vi "UHR-Fleezers Control (host) - 12.3.1.vi"() -> ()   [LabVIEW 2012] (continued)
  T20 = cluster{"New Image":T2, "New Image":T2, "New Image":T2, "New Image":T2, "New Image":T2}
  T21 = typedef "XDNodeRunTimeDep.lvlib/timing_clust.ctl" = cluster{"Expected End [f-1]":u64, "Actual End [f-1]":u64, "Finished Late? [f-1]":bool, "Expected End [i-1]":u64, "Actual End [i-1]":u64, "Finished Late? [i-1]":bool, "Expected Start [i]":u64, "Actual Start [i]":u64, "Expected Start [f]":u64, "Actual Start [f]":u64, "Source Name":string, "Structure Name":string, "Period":i64, "Deadline":i64, "Offset":i64, "Start":i64, "Priority":i32, "Timeout":i32, "Mode":T22, "Wakeup Reason":T23, "Error":errorcluster, "Source Type":string, "Secondary Source Type":string, "Global End Time":u64, "Global Start Time":u64, "Frame Duration":u64, "Iteration Duration":u64, "Assigned CPU":i32, "I/O Scan Engine Mode":u32}
  T22 = typedef "XDNodeRunTimeDep.lvlib/nitl_modes.ctl" = enum32{"No Change", "Process missed periods, maintain original phase", "Discard missed periods, maintain original phase", "Process missed periods, ignore original phase", "Discard missed periods, ignore original phase"}
  T23 = typedef "XDNodeRunTimeDep.lvlib/wakeup.ctl" = enum32{"Normal", "Aborted", "Asynchronous wakeup", "Timing source error", "Timed loop error", "Timeout"}
  T24 = enum32{"Status", "Sample Stage", "Syringe Pump", "Trap Control (RF)", "APD Counting", "Fluorescence Laser Control", "Trap AI", "Video", "FPGA"}
  T25 = enum16{"big-endian, network order", "native, host order", "little-endian"}
  T26 = enum16{"open", "replace", "create", "open or create", "replace or create", "replace or create with confirmation"}
  T27 = cluster{"Scan Range AOD (nm) 2":dbl, "Step Size AOD (nm) 2":dbl, "Scan Speed AOD (nm/s) 2":dbl, "Number of scans (AOD) 2":u16, "Label":string}
  T28 = cluster{"[0]":dbl, "[1]":dbl, "[2]":dbl, "[3]":dbl, "[4]":dbl, "[5]":dbl}
  T29 = cluster{"Diameter (mm)":dbl, "Units":dbl, "Volume":dbl, "Rate":dbl}
  T30 = cluster{"Left":i32, "Top":i32, "Width":u32, "Height":u32}
  T31 = cluster{cluster{"Left":i32, "Top":i32, "Width":u32, "Height":u32}}[]
  T32 = enum32{"Normal Display", "Dual Display (APD)", "FFT", "High Res Display"}
  T33 = cluster{"Origin Pixel":cluster{"X":sgl, "Y":sgl}, "Angle Relative to Horizontal (deg)":sgl, "Axis Reference":u32}
  T34 = typedef "Simple Grid Descriptor" = cluster{"X Step":sgl, "Y Step":sgl, "Unit":T35}
  T35 = typedef "Image Unit" = enum32{"Undefined", "Angström", "Micrometer", "Millimeter", "Centimeter", "Meter", "Kilometer", "Microinch", "Inch", "Feet", "Nautical miles", "Standard miles", "Steps"}
  T36 = cluster{"averaging mode":u16, "weighting mode":u16, "number of averages":u32}
  T37 = cluster{"dB On (F)":bool, "unwrap phase (F)":bool, "convert to degree (F)":bool}
  T38 = cluster{string, string, string, string, string, string, string, string}
  T39 = cluster{string, string, string, string, string, string, string, string, string, string, string, string}
  T40 = cluster{string, string, string, string, string, string, string, string, string, string, string, string, string}
  T41 = cluster{string, string, string, string, string, string, string, string, string, string, string, string, string, string}
  T42 = cluster{"BD 1 Frequency 1 (MHz)":dbl, "BD 1 Frequency 2 (MHz)":dbl}
  T43 = cluster{"f0":dbl, "df":dbl, "magnitude":dbl[]}[][]
  T44 = enum32{"setting", "request", "request control", "info", "statistics", "system settings", "I/O sub system", "HRT control", "camera descriptions", "device specific data", "event sub system settings", "event sub system results", "image memory manager"}
  T45 = typedef "AviRefnum.ctl" = refnum<k1>
  T46 = typedef "imagedata.ctl" = cluster{"image type":i32, "image depth":i32, "image":u8[], "mask":u8[], "colors":u32[], "Rectangle":cluster{"left":i16, "top":i16, "right":i16, "bottom":i16}}
diagram:
  w69 = u16 20 items=["1.0"=10, "1.5"=15, "2.0"=20] ("stop bits (10: 1 bit)")
  w72 = u16 20 items=["1.0"=10, "1.5"=15, "2.0"=20] ("stop bits (10: 1 bit)")
  w98 = u16 20 items=["1.0"=10, "1.5"=15, "2.0"=20] ("stop bits (10: 1 bit)")
  w4 = T17 2 items=["Grayscale (U8)", "Grayscale (I16)", "Grayscale (SGL)", "Complex (CSG)", "RGB (U32)", "HSL (U32)", "RGB (U64)", "Grayscale (U16)"] ("Image Type")
  w228 = 10.0 ("y")
  w227 = 32767.0 ("y")
  w243 = 6.0  # clock mult.
  w244 = 49152000.0  # TCXO frequ.
  # "What are these?"
  # "I don't think you need to do this.\nEverytime you want to adjust phase you always set this anyway.\nSince we removed the separate +/- controls.\n\nHaven't added for added fl lasers.  Should remove this code."
  # "Bottom 1 Harvard"
  # "Top 3 Harvard"
  # "Center Harvard"
  # "Bottom 1 Harvard"
  # "Top 3 Harvard"
  # "Center Harvard"
  n1 = Build Array("DIO count 1 (ticks)", "DIO count 2 (ticks)", "DIO count 3 (ticks)") -> (w149:u16[])
  n2 = xnode "Open FPGA VI Reference"("resource name"=T18 "750kHzDAQ") -> ("FPGA VI Reference Out"=w252:T19, "error out"=w251:errorcluster)  [unwired: 1 in]
  n3 = local read "AO1"() -> (w222:dbl)
  n4 = local read "AO2"() -> (w221:dbl)
  n5 = local read "Scan Increment (MHz)"() -> (w239:dbl)
  n6 = local read "Continuous MCL Scanning"() -> (w209:bool)
  n7 = local read "Fast Scan Dir"() -> (w208:bool)
  n8 = xnode "Invoke Method"("FPGA VI Reference In"=w252, "error in"=w251) -> ("FPGA VI Reference Out"=w8:T19, "error out"=w168:errorcluster)
  n9 = local read "Number of scans (MCL)"() -> (w210:u64)
  n10 = Multiply(x=w222, y=w227) -> (x*y=w224:dbl)
  n11 = Multiply(x=w221, y=w227) -> (x*y=w226:dbl)
  n12 = Divide(x=w224, y=w228) -> (x/y=w223:dbl)
  n13 = Divide(x=w226, y=w228) -> (x/y=w225:dbl)
  n14 = To Word Integer(number=w223) -> (16bit integer=w220:i16)
  n15 = To Word Integer(number=w225) -> (16bit integer=w219:i16)
  n16 = Not(x=w208) -> (.not. x?=w203:bool)
  n17 = local read "Cycles/step (MCL)"() -> (w211:u64)
  n18 = Multiply(x=w239, y=1000.0) -> (x*y=w246:dbl)
  n19 = local read "Scan steps (MCL)"() -> (w212:u64)
  n20 = local read "Desired Scan Incr (V)"() -> (w214:dbl)
  n21 = Scale By Power Of 2(n=48, x=w246) -> (x*2^n=w247:dbl)
  n22 = Unbundle By Name(cluster{"output high":i16, "output low":i16} {"output high"=3000, "output low"=0} ("FB output range 1")) -> ("output high"=w50:i16, "output low"=w49:i16)
  n23 = Multiply(x=w244, y=w243) -> (x*y=w242:dbl)
  n24 = Divide(x=w247, y=w242) -> (x/y=w241:dbl)
  n25 = local read "Setpoints (V)"() -> (w258:cluster{"Set 1":dbl, "Set 2":dbl})
  n26 = To Quad Integer(1:w241) -> (0:w238:i64)
  n27 = Divide(x=40000000.0, y="AI Count (ticks)") -> (x/y=w199:dbl)
  n28 = Multiply(x=w214, y=32767.0) -> (x*y=w216:dbl)
  n29 = local read "Trap Intensity PID Gains"() -> (w253:T9)
  n30 = local write "Trap Pos FIFO Timeout"(u16 0 ("Trap Pos FIFO Timeout")) -> ()
  n31 = local read "Number Interlace Sets"() -> (w142:u8)
  n32 = Split 1D Array(array=w149, index=w142) -> (first subarray=w151:u16[])  [unwired: 1 out]
  n33 = Add Array Elements(numeric array=w151) -> (sum=w150:u16)
  n34 = local read "# Samples/channel"() -> (w231:u32)
  n35 = local read "Number of F/B Scans (AOD)"() -> (w232:u16)
  n36 = local read "Not-Interlacing Set"() -> (w141:enum32{"Set 1", "Set 2", "Set 3"})
  n37 = To Unsigned Byte Integer(number=w141) -> (unsigned 8bit integer=w147:u8)
  n38 = Index Array(array=w149, index=w147) -> (element=w148:u16)
  n39 = local read "Feedback On/Off"() -> (w261:cluster{"Set 1":bool, "Set 2":bool})
  n40 = local read "Scan steps (AOD)"() -> (w237:u64)
  n41 = local read "All FB On/Off"() -> (w262:bool)
  n42 = local read "Cycles/step (AOD)"() -> (w236:u64)
  n43 = local write "AI rate (Hz)"(w199) -> ()
  n44 = Divide(x=w216, y=10.0) -> (x/y=w215:dbl)
  n45 = Multiply(x=w237, y=w236) -> (x*y=w235:u64)
  n46 = Unbundle By Name(w253) -> ("proportional gain (Kc)"=w54:i16, "integral gain (Kc*Ts/Ti)"=w53:i16, "derivative gain (Kc*Td/Ts)"=w52:i16)
  n47 = property on="AI Count (ticks)" class="DigNum (strict)"("Val(Sgnl)"="AI Count (ticks)") -> ()  [unwired: 2 in, 2 out]
  n48 = Multiply(x=3276.7, y=w258) -> (x*y=w257:cluster{"Set 1":dbl, "Set 2":dbl})
  n49 = To Word Integer(number=w215) -> (16bit integer=w213:i16)
  n50 = Multiply(x=w235, y=u64 2) -> (x*y=w233:u64)
  n51 = Divide(x=w199, y="FPGA Ave.") -> (x/y=w200:dbl)
  n52 = To Word Integer(number=w257) -> (16bit integer=w256:cluster{"Set 1":i16, "Set 2":i16})
  n53 = Multiply(x=w233, y=w232) -> (x*y=w230:u64)
  n54 = local read "Sets to FIFO (Traps)"() -> (w58:T15)
  n55 = local write "Ave. Rate (Hz)"(w200) -> ()
  n56 = Divide(x=w230, y=w231) -> (x/y=w229:dbl)
  n57 = Unbundle By Name(w256) -> ("Set 1"=w255:i16, "Set 2"=w254:i16)
  n58 = local read "2D or 1D Scan"() -> (w160:bool)
  n59 = local write "Data points/scans"(w230) -> ()
  n60 = local read "Scan BD"() -> (w248:bool)
  n61 = And(x=w261, y=w262) -> (x .and. y?=w260:cluster{"Set 1":bool, "Set 2":bool})
  n62 = local write "Data points/scan (f/b)"(w233) -> ()
  n63 = Reciprocal(x=w200) -> (1/x=w201:dbl)
  n64 = local read "N Acq Sets (Traps + Fl.)"() -> (w192:i16)
  n65 = local write "N sets should be saved"(w229) -> ()
  n66 = Unbundle By Name(w260) -> ("Set 1"=w264:bool, "Set 2"=w263:bool)
  n67 = local read "Interlace"() -> (w143:bool)
  n68 = Select(t=w150, s=w143, f=w148) -> (s? t:f=w140:u16)
  n69 = local write "Update Count (MCL)"(w140) -> ()
  n70 = local write "Total Counts (ticks)"(w140) -> ()
  n71 = local write "Ave. Period (s)"(w201) -> ()
  n72 = Unbundle By Name(w58) -> ("Set 1"=w57:bool, "Set 2"=w56:bool, "Set 3"=w55:bool)
  n73 = property on="2D or 1D Scan" class="Bool (strict)"("Val(Sgnl)"=w160) -> ()  [unwired: 2 in, 2 out]
  n74 = xnode "Read/Write Control"("FPGA VI Reference In"=w159, "error in"=w168, "ai count"="AI Count (ticks)", "Interlace ON/OFF"=w143, "Number Interlace Cycles"=w142, "Set 1"=w57, "Set 2"=w56, "Set 3"=w55, "FB On/Off Set 1"=w264, "FB On/Off Set 2"=w263, "Interlace Off Parameters"=w141, "FB Setpoint Set 1"=w255, "FB Setpoint Set 2"=w254, "P1"=w54, "I1"=w53, "D1"=w52, "FB1 output high"=w50, "FB1 output low"=w49, "Cycles per step"=w236, "Scan BD"=w248, "Number of scans"=w232, "Scan steps"=w237, "Scan freq.  increment"=w238, "AO1"=w220, "AO2"=w219, "Scan freq.  increment (MCL)"=w213, "Scan steps (MCL)"=w212, "Cycles per step (MCL)"=w211, "Number of scans (MCL)"=w210, "MCL count"=w140, "Cont. Scan (MCL)"=w209, "MCL Scan Axis"=w203, "1D or 2D Scan?"=w160, "N of AI1 Int Acq Sets"=w192, "Amp switch delay"="Amp switch delay", "Swap F1 and F2"="Swap F1 and F2", "APD to FIFO"=FALSE, "DIO count 1 (ticks)"="DIO count 1 (ticks)", "DIO count 2 (ticks)"="DIO count 2 (ticks)", "DIO count 3 (ticks)"="DIO count 3 (ticks)") -> ("FPGA VI Reference Out"=w10:T19, "error out"=w9:errorcluster)  [unwired: 1 in]
  n75 = local read "Laser interlacing mode"() -> (w139:enum32{"Laser ON", "Laser OFF", "Interlace"})
  n76 = local read "Green Laser ON"() -> (w138:bool)
  n77 = local read "Trap Pos. FB Range"() -> (w48:T12)
  n78 = local read "Trap Pos. FB Gains"() -> (w47:T11)
  n79 = Multiply(x="Green Intensity - FB OFF (%)", y=655.35) -> (x*y=w131:dbl)
  n80 = local read "Invert laser interlacing"() -> (w25:bool)
  n81 = local read "Trap Pos. AI1 X Pre-scale"() -> (w86:u16)
  n82 = Multiply(x="Green FB Setpoint (mV)", y=3.2767) -> (x*y=w128:dbl)
  n83 = local read "Trap Pos FB Int Count"() -> (w80:u16)
  n84 = local read "Differential FB?"() -> (w74:bool)
  n85 = local read "Neg. TTrig FPGA"() -> (w76:bool)
  n86 = Multiply(x="Red FB Setpoint (mV)", y=3.2767) -> (x*y=w34:dbl)
  n87 = To Unsigned Word Integer(number=w131) -> (unsigned 16bit integer=w129:u16)
  n88 = Multiply(x="Red Intensity - FB OFF (%)", y=655.35) -> (x*y=w30:dbl)
  n89 = To Word Integer(number=w128) -> (16bit integer=w126:i16)
  n90 = Unbundle By Name("Green FB Gains") -> ("proportional gain (Kc)"=w39:i16, "integral gain (Kc*Ts/Ti)"=w38:i16, "derivative gain (Kc*Td/Ts)"=w37:i16)
  n91 = case shown="False" w138 {
    tunnel: w139 -> [_ w290]
    tunnel: [enum32{"Laser ON", "Laser OFF", "Interlace"}."Laser OFF" ("Green laser mode") w290] -> w24
    frame False {
    }
    frame True {
    }
  }
  n92 = To Word Integer(number=w34) -> (16bit integer=w31:i16)
  n93 = Unbundle By Name("Red FB Gains") -> ("proportional gain (Kc)"=w22:i16, "integral gain (Kc*Ts/Ti)"=w21:i16, "derivative gain (Kc*Td/Ts)"=w20:i16)
  n94 = Unbundle By Name(w47) -> ("proportional gain (Kc)"=w43:fxp<+/-,16,8>, "integral gain (Kc*Ts/Ti)"=w42:fxp<+/-,16,8>, "derivative gain (Kc*Td/Ts)"=w41:fxp<+/-,16,8>)
  n95 = To Unsigned Word Integer(number=w30) -> (unsigned 16bit integer=w27:u16)
  n96 = Unbundle By Name(w48) -> ("output high"=w46:fxp<+/-,16,1>, "output low"=w44:fxp<+/-,16,1>)
  n97 = local read "Trap Pos FB Monitor\nT1 or T2"() -> (w91:bool)
  n98 = local read "Trap Pos FB Negate Action"() -> (w90:bool)
  n99 = local read "Trap Pos. FB Offset Factor"() -> (w89:i64)
  n100 = local read "Trap Pos. FB Mult Factor"() -> (w88:i64)
  n101 = xnode "Read/Write Control"("FPGA VI Reference In"=w10, "error in"=w9, "Invert GI 2"=w25, "Operating Mode 2"=w24, "P3"=w39, "I3"=w38, "D3"=w37, "Green FB Setpoint"=w126, "Green FB On/Off"="Green FB On/Off", "Current Out"=w129, "Green int current ON count adj"="Green int current ON count adj", "Operating Mode"=w24, "Invert GI"=w25, "Trap Pos FB Monitor T1 or T2"=w91, "Trap Pos FB Negate Action"=w90, "Trap Pos. FB Offset Factor"=w89, "Trap Pos. FB Mult Factor"=w88, "Force feedback"=FALSE, "AI1 X Scale"=w86, "Trap Pos to FIFO"=TRUE, "Trap Pos FB Int Count"=w80, "TTrig Negate Pos"=w76, "FB Trig Integrate"="FB Trig Integrate", "Diff FB Measurement?"=w74, "Negate Diff?"="Negate Diff?", "P2"=w43, "I2"=w42, "D2"=w41, "FB2 output high"=w46, "FB2 output low"=w44, "Red FB Setpoint"=w31, "RI Current Out"=w27, "Red int current ON count adj"="Red int current ON count adj", "Red Laser Operating Mode"=w24, "RI Operating Mode 2"=w24, "Invert RI 2"=w25, "Invert RI"=w25, "P4"=w22, "I4"=w21, "D4"=w20, "Red FB On/Off"="Red FB On/Off") -> ("FPGA VI Reference Out"=w15:T19, "error out"=w17:errorcluster)
  n102 = stacked-sequence {
    tunnel: w17 -> [_ _ w298]
    tunnel: [_ _ w298] -> w16
    tunnel: w15 -> [_ _ w299]
    tunnel: [_ _ w299] -> w14
    frame #0 {
      # "APD loop counts"
      # "Fluorescence loop counts (rates)"
      n103 = local read "APD Integration Time (s)"() -> (w292:dbl)
      n104 = local read "Interlace ON count"() -> (w293:u16)
      n105 = property on="APD Integration Time (s)" class="DigNum (strict)"("Val(Sgnl)"=w292) -> ()  [unwired: 2 in, 2 out]
      n106 = property on="Interlace ON count" class="DigNum (strict)"("Val(Sgnl)"=w293) -> ()  [unwired: 2 in, 2 out]
      "Number of APDs" <- 3.0 ("Number of APDs")
    }
    frame #1 {
      # "Number of APDs affects\nAPD DMA transfer"
      # "General settings for all lasers:"
      # "And includes all laser\nON/OFF settings"
      # "Fluorescent lasers settings:"
      # "Blue laser settings:"
      n107 = local read "Laser interlacing mode"() -> (w295:enum32{"Laser ON", "Laser OFF", "Interlace"})
      n108 = local read "Invert laser interlacing"() -> (w294:bool)
      n109 = local read "Blue FB On/Off"() -> (w296:bool)
      n110 = property on="Blue FB On/Off" class="Bool (strict)"("Val(Sgnl)"=w296) -> ()  [unwired: 2 in, 2 out]
      n111 = property on="Invert laser interlacing" class="Bool (strict)"("Val(Sgnl)"=w294) -> ()  [unwired: 2 in, 2 out]
      n112 = property on="Laser interlacing mode" class="RadioBtnsControl (strict)"("Val(Sgnl)"=w295) -> ()  [unwired: 2 in, 2 out]
    }
    frame #2 {
      n113 = Wait (ms)(milliseconds to wait=u32 1000) -> ()  [unwired: 1 out]
    }
  }
  n114 = local write "Offset (nm)"(0.0 ("Offset (nm)")) -> ()
  n115 = local write "Bead Mean (nm)"(0.0 ("Bead Mean (nm)")) -> ()
  n116 = xnode "Invoke Method"("FPGA VI Reference In"=w14, "error in"=w16, "Requested Depth"="Trap AI FIFO Depth") -> ("FPGA VI Reference Out"=w94:T19, "error out"=w93:errorcluster)  [unwired: 1 out]
  n117 = xnode "Invoke Method"("FPGA VI Reference In"=w94, "error in"=w93, "Requested Depth"="Trap Position FIFO Depth") -> ("FPGA VI Reference Out"=w82:T19, "error out"=w81:errorcluster)  [unwired: 1 out]
  n118 = flat-sequence "Safety limits on RF frequencies and amplitudes (for AOM protection)" {
    tunnel: w8 -> [w304]
    tunnel: [w304] -> w159
    tunnel: [w303] -> w158
    tunnel: [w302] -> w157
    tunnel: [w300] -> w155
    tunnel: [w301] -> w156
    frame #0 {
      w301 = T16 {"Minimum"=0.0, "Maximum"=40.0, "Increment"=1.0} ("Min Max Inc")
      w300 = T16 {"Minimum"=0.0, "Maximum"=50.0, "Increment"=1.0} ("Data Entry Limits")
      w303 = T16 {"Minimum"=60.0, "Maximum"=90.0, "Increment"=1.0} ("Min Max Inc")
      w302 = T16 {"Minimum"=0.0, "Maximum"=50.0, "Increment"=1.0} ("Data Entry Limits")
      n119 = property on="BD 2 Frequency 1 (MHz)" class="DigNum (strict)"("Data Range"=w301) -> ()  [unwired: 2 in, 2 out]
      n120 = property on="BD 2 Frequency 3 (MHz)" class="DigNum (strict)"("Data Range"=w301) -> ()  [unwired: 2 in, 2 out]
      n121 = property on="BD 2 Frequency 2 (MHz)" class="DigNum (strict)"("Data Range"=w301) -> ()  [unwired: 2 in, 2 out]
      n122 = property on="BD 1 Frequency 1 (MHz)" class="DigNum (strict)"("Data Range"=w303) -> ()  [unwired: 2 in, 2 out]
      n123 = property on="BD 1 Frequency 2 (MHz)" class="DigNum (strict)"("Data Range"=w303) -> ()  [unwired: 2 in, 2 out]
      n124 = property on="BD 1 Frequency 3 (MHz)" class="DigNum (strict)"("Data Range"=w303) -> ()  [unwired: 2 in, 2 out]
      n125 = property on="BD 2 Amplitude 1 (%)" class="DigNum (strict)"("Data Range"=w300) -> ()  [unwired: 2 in, 2 out]
      n126 = property on="BD 2 Amplitude 2 (%)" class="DigNum (strict)"("Data Range"=w300) -> ()  [unwired: 2 in, 2 out]
      n127 = property on="BD 2 Amplitude 3 (%)" class="DigNum (strict)"("Data Range"=w300) -> ()  [unwired: 2 in, 2 out]
      n128 = property on="BD 1 Amplitude 3 (%)" class="DigNum (strict)"("Data Range"=w302) -> ()  [unwired: 2 in, 2 out]
      n129 = property on="BD 1 Amplitude 2 (%)" class="DigNum (strict)"("Data Range"=w302) -> ()  [unwired: 2 in, 2 out]
      n130 = property on="BD 1 Amplitude 1 (%)" class="DigNum (strict)"("Data Range"=w302) -> ()  [unwired: 2 in, 2 out]
      "X RF Frequency Limits (MHz)" <- w303
      "X RF Amplitude Limits (%)" <- w302
      "Y RF Amplitude Limits (%)" <- w300
      "Y RF Frequency Limits (MHz)" <- w301
    }
  }
  n131 = xnode "Invoke Method"("FPGA VI Reference In"=w82, "error in"=w81) -> ("FPGA VI Reference Out"=w167:T19, "error out"=w166:errorcluster)  [unwired: 1 in]
  n132 = flat-sequence "Initial FPGA Loop Relative Phase Adjustment" {
    tunnel: "Initial Phase Adjustment (AI1)" -> [w322]
    tunnel: "Initial Phase Adjustment (GI)" -> [w321]
    tunnel: w167 -> [w320]
    tunnel: w166 -> [w319]
    tunnel: "Initial Phase Adj. (MCL)" -> [w318]
    tunnel: [w323] -> w176
    tunnel: [w317] -> w172
    tunnel: "Initial Phase Adjustment (APD Acq)" -> [w316]
    tunnel: "Initial Phase Adjustment (APD 1 Gate)" -> [w315]
    tunnel: "Initial Phase Adjustment (Green FB)" -> [w314]
    tunnel: "Initial Phase Adjustment (GI) 2" -> [w313]
    tunnel: "Initial Phase Adjustment (APD 2 Gate)" -> [w312]
    tunnel: "Initial Phase Adjustment (RI)" -> [w311]
    tunnel: "Initial Phase Adjustment (RI) 2" -> [w310]
    tunnel: "Initial Phase Adjustment (RI FB)" -> [w309]
    tunnel: "Initial Phase Adjustment (BI DO)" -> [w308]
    tunnel: "Initial Phase Adjustment (BI AO)" -> [w307]
    tunnel: "Initial Phase Adjustment (BI AI)" -> [w306]
    tunnel: "Initial Phase Adjustment (APD 3 Gate)" -> [w305]
    tunnel: w176 -> [w325]
    tunnel: [w326] -> w173
    tunnel: w172 -> [w326]
    tunnel: [w325] -> w171
    tunnel: w173 -> [w329]
    tunnel: w171 -> [w328]
    tunnel: [w331] -> w170
    tunnel: [w330] -> w169
    tunnel: [w333] -> w174
    tunnel: [w334] -> w175
    tunnel: w170 -> [w334]
    tunnel: w169 -> [w333]
    frame #0 {
      n133 = xnode "Read/Write Control"("FPGA VI Reference In"=w320, "error in"=w319, "Phase count adjustment"=w322, "Phase count adjustment (GI)"=w321, "Phase count adjustment (MCL)"=w318, "Phase Count Adjustment (APD Acq)"=w316, "Phase count adjustment (APD 1 Gate)"=w315, "Phase count adjustment (APD 2 Gate)"=w312, "Phase count adjustment (Green FB)"=w314, "Phase count adjustment (GI) 2"=w313, "Phase count adjustment (RI)"=w311, "Phase count adjustment (RI) 2"=w310, "Phase count adjustment (Red FB)"=w309, "Phase count adjustment (BI AO)"=w307, "Phase count adjustment (BI D)"=w308, "Phase count adjustment (Blue Int)"=w306, "Phase count adjustment (APD 3 Gate)"=w305) -> ("FPGA VI Reference Out"=w317:T19, "error out"=w323:errorcluster)
    }
    frame #1 {
      n134 = Wait (ms)(milliseconds to wait=u32 100) -> ()  [unwired: 1 out]
    }
    frame #2 {
      w327 = TRUE
      n135 = xnode "Read/Write Control"("FPGA VI Reference In"=w329, "error in"=w328, "+ phase"=w327, "+ phase (GI)"=w327, "+ phase (MCL)"=w327, "+ phase (APD Acq)"=w327, "+ phase (APD 1 Gate)"=w327, "+ phase (APD 2 Gate)"=w327, "+ phase (Green FB)"=w327, "+ phase (GI) 2"=w327, "+ phase (RI)"=w327, "+ phase (RI) 2"=w327, "+ phase (BI AO)"=w327, "+ phase (BI D)"=w327, "+ phase (Blue Int)"=w327, "+ phase (APD 3 Gate)"=w327) -> ("FPGA VI Reference Out"=w330:T19, "error out"=w331:errorcluster)
    }
    frame #3 {
      n136 = Wait (ms)(milliseconds to wait=u32 100) -> ()  [unwired: 1 out]
    }
  }
  n137 = local read "Phase adj. (Green FB)"() -> (w152:i16)
  n138 = local read "Phase adj. (GI) 2"() -> (w132:i16)
  n139 = local read "Phase adjust (MCL)"() -> (w204:i16)
  n140 = local read "Phase adj. (AI1)"() -> (w206:i16)
  n141 = local read "Phase adj. (GI)"() -> (w205:i16)
  n142 = xnode "Read/Write Control"("FPGA VI Reference In"=w174, "error in"=w175, "Phase count adjustment"=w206, "Phase count adjustment (GI)"=w205, "Phase count adjustment (MCL)"=w204, "Phase Count Adjustment (APD Acq)"="Phase Adj. (APD Acq)", "Phase count adjustment (APD 1 Gate)"="Phase Adj. (APD 1 Gate)", "Phase count adjustment (APD 2 Gate)"="Phase Adj. (APD 2 Gate)", "Phase count adjustment (Green FB)"=w152, "Phase count adjustment (GI) 2"=w132) -> ("FPGA VI Reference Out"=w118:T19, "error out"=w181:errorcluster)
  n143 = call "Initialize RF boards - interlace 3.vi"("error in"=w181, "FPGA VI Reference In"=w118) -> ("error out"=w179:errorcluster, "FPGA VI Reference Out"=w180:T19)
  n144 = call "set RF board frequency - interlace.vi"("Board 2 Frequency Limits"=w156, "Board 1 Frequency Limits"=w158, "error in"=w179, "FPGA VI Reference In"=w180, "Board 2 Frequency 3 (MHz)"="BD 2 Frequency 3 (MHz)", "Board 1 Frequency 3 (MHz)"="BD 1 Frequency 3 (MHz)", "Board 2 Frequency 2 (MHz)"="BD 2 Frequency 2 (MHz)", "Board 2 Frequency 1 (MHz)"="BD 2 Frequency 1 (MHz)", "Board 1 Frequency 2 (MHz)"="BD 1 Frequency 2 (MHz)", "Board 1 Frequency 1  (MHz)"="BD 1 Frequency 1 (MHz)") -> ("error out"=w279:errorcluster, "FPGA VI Reference Out"=w280:T19)
  n145 = call "set RF board amplitude - interlace.vi"("Board 2 Amplitude Limits"=w155, "Board 1 Amplitude Limits"=w157, "error in"=w279, "FPGA VI Reference In"=w280, "Board 2 Amplitude 3 (%)"="BD 2 Amplitude 3 (%)", "Board 1 Amplitude 3 (%)"="BD 1 Amplitude 3 (%)", "Board 2 Amplitude 2 (%)"="BD 2 Amplitude 2 (%)", "Board 2 Amplitude 1 (%)"="BD 2 Amplitude 1 (%)", "Board 1 Amplitude 2 (%)"="BD 1 Amplitude 2 (%)", "Board 1 Amplitude 1 (%)"="BD 1 Amplitude 1 (%)") -> ("error out"=w267:errorcluster, "FPGA VI Reference Out"=w268:T19)
  n146 = flat-sequence {
    tunnel: w268 -> [w344]
    tunnel: w267 -> [w343]
    tunnel: [w342] -> w272
    tunnel: [w341] -> w271
    tunnel: [w348] -> w270
    tunnel: w272 -> [w348]
    tunnel: [w347] -> w269
    tunnel: w271 -> [w347]
    tunnel: w270 -> [w357]
    tunnel: w269 -> [w356]
    tunnel: [w355] -> w7
    tunnel: [w354] -> w83
    frame #0 {
      w335 = FALSE ("Retract Pump 3")
      n147 = local read "Trap 1 (ON/OFF)"() -> (w336:bool)
      n148 = xnode "Read/Write Control"("FPGA VI Reference In"=w344, "error in"=w343, "Direct RF Box  Communication"=FALSE) -> ("FPGA VI Reference Out"=w342:T19, "error out"=w341:errorcluster)
      n149 = local write "Saving..."(FALSE ("Saving Data")) -> ()
      n150 = local write "Stop All"(FALSE ("Stop All")) -> ()
      n151 = local write "Retract Pump 1"(w335) -> ()
      n152 = local write "Retract Pump 3"(w335) -> ()
      n153 = local write "Index"(1.0 ("Index")) -> ()
      n154 = property on="Trap 1 ON" class="Bool (strict)"("Value"=w336) -> ()  [unwired: 2 in, 2 out]
      "Manipulating Trap" <- FALSE ("Manipulating Trap")
    }
    frame #1 {
      n155 = local read "Trap 2 (ON/OFF)"() -> (w346:bool)
      n156 = Wait (ms)(milliseconds to wait=u32 10) -> ()  [unwired: 1 out]
      n157 = property on="Trap 2 ON" class="Bool (strict)"("Val(Sgnl)"=w346) -> ()  [unwired: 2 in, 2 out]
    }
    frame #2 {
      n158 = local read "Scan Range (nm)"() -> (w350:dbl)
      n159 = xnode "Read/Write Control"("FPGA VI Reference In"=w357, "error in"=w356, "FPGA Controls  RF Box"=TRUE ("Direct RF Box  Communication")) -> ("FPGA VI Reference Out"=w355:T19, "error out"=w354:errorcluster)
      n160 = call "Update messages.vi"("Message to add"="UHR-Fleezers ready.", "Old message string"="") -> ("New message string"=w353:string)
      n161 = local write "Messages"(w353) -> ()
      n162 = property on="Scan Range (nm)" class="DigNum (strict)"("Val(Sgnl)"=w350) -> ()  [unwired: 2 in, 2 out]
    }
  }
  n163 = Subtract(x="BD 1 Frequency 1 (MHz)", y="BD 1 Frequency 2 (MHz)") -> (x-y=w191:dbl)
  n164 = Subtract(x="BD 2 Frequency 1 (MHz)", y="BD 2 Frequency 2 (MHz)") -> (x-y=w190:dbl)
  n165 = Square(x=w190) -> (x^2=w188:dbl)
  n166 = Square(x=w191) -> (x^2=w189:dbl)
  n167 = Add(x=w189, y=w188) -> (x+y=w187:dbl)
  n168 = Square Root(x=w187) -> (sqrt(x)=w186:dbl)
  n169 = local write "Trap Delta (MHz)"(w186) -> ()
  n170 = call-poly "VISA Configure Serial Port"("VISA resource name"="Bottom  1 Harvard Syringe Pump Serial Port", "baud rate (9600)"=u32 115200, "stop bits (10: 1 bit)"=w69) -> ("VISA resource name out"=w65:refnum<visa-resource-name>, "error out"=w64:errorcluster)  [unwired: 4 in, 7 out]
  n171 = call-poly "VISA Configure Serial Port"("VISA resource name"="Top 3 Harvard Syringe Pump Serial Port", "baud rate (9600)"=u32 115200, "stop bits (10: 1 bit)"=w72) -> ("VISA resource name out"=w67:refnum<visa-resource-name>, "error out"=w66:errorcluster)  [unwired: 4 in, 7 out]
  n172 = call-poly "VISA Configure Serial Port"("VISA resource name"="Sample Chamber Stage Serial Port") -> ("VISA resource name out"=w113:refnum<visa-resource-name>, "error out"=w114:errorcluster)  [unwired: 5 in, 8 out]
  "Stage Control Serial Error" <- w114
  n173 = call-poly "VISA Configure Serial Port"("VISA resource name"="Center Harvard Syringe Pump Serial Port", "baud rate (9600)"=u32 115200, "stop bits (10: 1 bit)"=w98) -> ("VISA resource name out"=w95:refnum<visa-resource-name>, "error out"=w96:errorcluster)  [unwired: 4 in, 7 out]
  n174 = call "IMAQ Create"("Image Name"="APD 1 Image", "Image Type"=w4) -> ("New Image"=w104:T2)  [unwired: 3 in, 1 out]
  n175 = call "IMAQ Create"("Image Name"="APD 2 Image", "Image Type"=w4) -> ("New Image"=w103:T2)  [unwired: 3 in, 1 out]
  n176 = call "IMAQ Create"("Image Name"="APD 3 Image", "Image Type"=w4) -> ("New Image"=w3:T2)  [unwired: 3 in, 1 out]
  n177 = call "IMAQ Create"("Image Name"="Det. X Image", "Image Type"=w4) -> ("New Image"=w102:T2)  [unwired: 3 in, 1 out]
  n178 = call "IMAQ Create"("Image Name"="Det. Y Image", "Image Type"=w4) -> ("New Image"=w101:T2)  [unwired: 3 in, 1 out]
  n179 = Bundle("New Image"=w104, "New Image"=w103, "New Image"=w3, "New Image"=w102, "New Image"=w101) -> (w100:T20)  [unwired: 1 in]
  n180 = node-c288(3 ("Processor")) -> (w120:T21)  [unwired: 3 out]
  n181 = node-c288() -> (w109:T21)  [unwired: 4 in]
  n182 = node-c288(2 ("Processor")) -> (w122:T21)  [unwired: 3 out]
  n183 = node-c288() -> (w124:T21)  [unwired: 4 out]
  n184 = node-c288(i64 1 ("Period"), 1 ("Processor")) -> (w195:T21)  [unwired: 2 out]
  n185 = node-c288() -> (w2:T21)  [unwired: 4 out]
  n186 = timed-loop "Oscillate Trap/AOM (fishing, conjugate plane alignment)" {
    tunnel: w8 -> [w360]
    tunnel: [w359] -> w125
    timing: w120 -> [_]
    timing-out: [_] -> w119
    stop <- w359 stop-if-true
    n187 = node-c288() -> ()  [unwired: 2 out]
    n188 = event shown="[1] \"Fl. Triggered...\": Value Change" {
      selector: _ -> [_ _ _]
      dyn-events: _ -> [_ _ _]
      timeout: _ -> [_ _ _]
      tunnel: w360 -> [w367 _ _]
      tunnel: [FALSE ("Stop All") _ w956] -> w359
      event "Oscillate Set 1", "Fish for Tether": Value Change {
        n189 = event-data() -> ()  [unwired: 6 out]
        n190 = local read "Oscillate Set 1"() -> (w366:bool)
        n191 = Or(x=w366, y="Fish for Tether") -> (x .or. y?=w364:bool)
        n192 = case shown="True" w364 {
          tunnel: w367 -> [_ w370]
          tunnel: "Fish for Tether" -> [_ w369]
          frame False {
          }
          frame True {
            n193 = case shown="True" w369 {
              selector: w369 -> [w373 w379]
              tunnel: [w373 w379] -> w368
              frame False {
              }
              frame True {
                n194 = local write "Scan axis 2"(TRUE) -> ()
                n195 = local write "Tether"(FALSE ("Tether")) -> ()
                n196 = local read "Flow ON during cal?"() -> (w374:bool)
                n197 = property on="Trap Delta (MHz)" class="DigNum (strict)"("Val(Sgnl)"="Furthest Delta (MHz)") -> ()  [unwired: 2 in, 2 out]
                n198 = Or(x="Flow ON during \nfishing?", y=w374) -> (x .or. y?=w375:bool)
                n199 = Wait (ms)(milliseconds to wait=u32 500) -> ()  [unwired: 1 out]
                n200 = property on="Sample Channel\nFlow" class="Bool (strict)"("Val(Sgnl)"=w375) -> ()  [unwired: 2 in, 2 out]
              }
            }
            n201 = node-c288() -> (w372:T21)  [unwired: 4 out]
            n202 = timed-loop "Oscillate AOD" {
              timing: w372 -> [_]
              timing-out: [_] -> w371
              tunnel: w370 -> [w389]
              tunnel: w368 -> [w382]
              i -> [w391]
              stop <- w388 stop-if-true
              n203 = node-c288() -> (w390:i64)  [unwired: 1 out]
              n204 = flat-sequence {
                tunnel: w391 -> [w418]
                tunnel: w390 -> [w417]
                tunnel: w389 -> [w396]
                tunnel: w382 -> [w399]
                tunnel: [w399] -> w387
                tunnel: [w398] -> w386
                tunnel: [w395] -> w385
                tunnel: [w392] -> w383
                tunnel: w387 -> [w454]
                tunnel: w386 -> [w452]
                tunnel: w385 -> [w451]
                tunnel: [w450] -> w384
                tunnel: w383 -> [w449]
                tunnel: [w526] -> w388
                tunnel: w384 -> [w525]
                frame #0 {
                  n205 = Divide(x=w417, y=i64 1000) -> (x/y=w412:dbl)
                  n206 = local read "BD 1 Frequency 2 (MHz)"() -> (w397:dbl)
                  n207 = Multiply(x="Osc. freq. (Hz)", y=6.283185307179586) -> (x*y=w415:dbl)
                  n208 = Multiply(x=w412, y=w418) -> (x*y=w414:dbl)
                  n209 = Multiply(x=w415, y=w414) -> (x*y=w394:dbl)
                  n210 = local read "BD 1 Frequency 1 (MHz)"() -> (w402:dbl)
                  n211 = local read "BD 2 Frequency 1 (MHz)"() -> (w401:dbl)
                  n212 = case shown="True" w399 {
                    tunnel: w394 -> [w424 w429]
                    tunnel: w402 -> [_ w440]
                    tunnel: w397 -> [_ w441]
                    tunnel: [w421 w435] -> w400
                    tunnel: [FALSE w432] -> w395
                    tunnel: [0.0 w425] -> w392
                    frame False {
                      n213 = Sine(x=w424) -> (sin(x)=w422:dbl)
                      n214 = Multiply(x=w422, y="Osc. amp. (MHz)") -> (x*y=w421:dbl)
                    }
                    frame True {
                      n215 = Cosine(x=w429) -> (cos(x)=w444:dbl)
                      n216 = Subtract(x=w441, y=w440) -> (x-y=w439:dbl)
                      n217 = Decrement(x=w444) -> (x-1=w443:dbl)
                      n218 = Subtract(x=w439, y="Closest Delta (MHz)") -> (x-y=w436:dbl)
                      n219 = Divide(x=w443, y=-2.0) -> (x/y=w437:dbl)
                      n220 = Multiply(x=w437, y=w436) -> (x*y=w435:dbl)
                      n221 = local read "Vec Mean of T1 T2"() -> (w431:dbl[])
                      n222 = Greater?(x=w431, y="Stop F (pN)") -> (0:w433:bool[])
                      n223 = Or Array Elements(Boolean array=w433) -> (logical OR=w432:bool)
                      n224 = Divide(x=w429, y=6.283185307179586) -> (x/y=w428:dbl)
                      n225 = Round Toward +Infinity(x=w428) -> (ceil(x): smallest int >= x=w425:dbl)
                      "Attempts" <- w425
                      n226 = Greater?(x=w425, y="Attempt Limit") -> (0:w427:bool)
                      n227 = case shown="True" w427 {
                        frame False {
                        }
                        frame True {
                          n228 = local write "Fish for Tether"(FALSE ("Fish for Tether")) -> ()
                          n229 = call <vilib>:"Beep.vi"() -> ()  [unwired: 3 in, 9 out]
                          n230 = local read "Messages"() -> (w446:string)
                          n231 = call "Update messages.vi"("Message to add"="Tether fishing timeout." ("Messages"), "Old message string"=w446) -> ("New message string"=→"Messages":string)
                        }
                      }
                    }
                  }
                  n232 = Select(t=w402, s="Scan axis 2", f=w401) -> (s? t:f=w405:dbl)
                  n233 = Add(x=w400, y=w405) -> (x+y=w398:dbl)
                  n234 = Select(t=w398, s="Scan axis 2", f=w402) -> (s? t:f=w408:dbl)
                  n235 = Select(t=w401, s="Scan axis 2", f=w398) -> (s? t:f=w407:dbl)
                  n236 = local read "Y RF Frequency Limits (MHz)"() -> (w403:T16)
                  n237 = local read "X RF Frequency Limits (MHz)"() -> (w404:T16)
                  n238 = local read "BD 1 Frequency 3 (MHz)"() -> (w411:dbl)
                  n239 = local read "BD 2 Frequency 2 (MHz)"() -> (w410:dbl)
                  n240 = local read "BD 2 Frequency 3 (MHz)"() -> (w409:dbl)
                  n241 = call "set RF board frequency - interlace.vi"("Board 2 Frequency Limits"=w403, "Board 1 Frequency Limits"=w404, "FPGA VI Reference In"=w396, "Board 2 Frequency 3 (MHz)"=w409, "Board 1 Frequency 3 (MHz)"=w411, "Board 2 Frequency 2 (MHz)"=w410, "Board 2 Frequency 1 (MHz)"=w407, "Board 1 Frequency 2 (MHz)"=w397, "Board 1 Frequency 1  (MHz)"=w408) -> ()  [unwired: 1 in, 2 out]
                }
                frame #1 {
                  n242 = And(x=w454, y=w451) -> (x .and. y?=w453:bool)
                  n243 = case "Only if were fishing and now formed tether" shown="False" w453 {
                    tunnel: w452 -> [w456 w471]
                    tunnel: [w455 w470] -> w450
                    tunnel: w449 -> [_ w466]
                    frame False {
                      n244 = local read "Fish for Tether"() -> (w455:bool)
                      n245 = case shown="False" w455 {
                        tunnel: w456 -> [w457 _]
                        frame False {
                          n246 = property on="BD 1 Frequency 1 (MHz)" class="DigNum (strict)"("Val(Sgnl)"=w457) -> ()  [unwired: 2 in, 2 out]
                        }
                        frame True {
                        }
                      }
                    }
                    frame True {
                      w470 = FALSE ("Fish for Tether")
                      n247 = call <vilib>:"Beep.vi"() -> ()  [unwired: 3 in, 9 out]
                      n248 = Number To Decimal String(number=w466, width (-)=i16 1) -> (decimal integer string=w464:string)
                      n249 = Concatenate Strings("Formed tether in ", w464, " attempt(s)." ("string")) -> (w461:string)
                      n250 = local read "Messages"() -> (w468:string)
                      n251 = local write "Fish for Tether"(w470) -> ()
                      n252 = call "Update messages.vi"("Message to add"=w461, "Old message string"=w468) -> ("New message string"=w467:string)
                      n253 = local write "Messages"(w467) -> ()
                      n254 = Get Date/Time In Seconds() -> (seconds since 1Jan1904=→"Time tether formed":timestamp)
                      n255 = local read "Flow ON during cal?"() -> (w458:bool)
                      n256 = property on="Sample Channel\nFlow" class="Bool (strict)"("Val(Sgnl)"=w458) -> (error out=w459:errorcluster)  [unwired: 2 in, 1 out]
                      n257 = case shown="\"2\", \"3\", \"4\", \"5\", \"6\"" "Then..." {
                        selector: "Then..." -> [_ w474]
                        tunnel: w471 -> [w473 _]
                        tunnel: w459 -> [_ _]
                        frame "1", Default {
                          n258 = property on="BD 1 Frequency 1 (MHz)" class="DigNum (strict)"("Val(Sgnl)"=w473) -> ()  [unwired: 2 in, 2 out]
                        }
                        frame "2", "3", "4", "5", "6" {
                          n259 = flat-sequence {
                            tunnel: w474 -> [w476]
                            frame #0 {
                              n260 = property on="Trap Delta (MHz)" class="DigNum (strict)"("Val(Sgnl)"="Move to Delta 1 (MHz)") -> ()  [unwired: 2 in, 2 out]
                            }
                            frame #1 {
                              n261 = case shown="\"5\", \"6\"" w476 {
                                selector: w476 -> [w479 w489 _]
                                frame "3", "4" {
                                n262 = flat-sequence {
                                tunnel: w479 -> [w480]
                                tunnel: [w480] -> w477
                                tunnel: [w482] -> w478
                                tunnel: w477 -> [w482]
                                tunnel: w478 -> [w486]
                                frame #0 {
                                n263 = property on="Green Laser ON" class="Bool (strict)"("Val(Sgnl)"=TRUE ("Value (Signaling)")) -> ()  [unwired: 2 in, 2 out]
                                }
                                frame #1 {
                                n264 = Multiply(x="Wait Before Save (s)", y=u32 1000 ("x")) -> (x*y=w484:u32)
                                n265 = Wait (ms)(milliseconds to wait=w484) -> ()  [unwired: 1 out]
                                }
                                frame #2 {
                                n266 = property on="Start Saving" class="Bool (strict)"("Value"=TRUE ("Start Saving")) -> ()  [unwired: 2 in, 2 out]
                                n267 = case shown="\"4\"" w486 {
                                frame Default {
                                }
                                frame "4" {
                                n268 = property on="Fl. Triggered..." class="Bool (strict)"("Val(Sgnl)"=TRUE ("Value (Signaling)")) -> ()  [unwired: 2 in, 2 out]
                                }
                                }
                                }
                                }
                                }
                                frame "5", "6" {
                                n269 = stacked-sequence {
                                tunnel: w489 -> [_ _ _ _ _ _ w501]
                                frame #0 {
                                n270 = Replace Array Subset(array=u32[] [0] ("Index Values"), new element="Raster Set Upon Tether", index=0) -> (w490:u32[])
                                n271 = property on="Saved AOD Raster Scan Parameter Sets" class="Arr (strict)"("Index Values"=w490) -> ()  [unwired: 2 in, 2 out]
                                }
                                frame #1 {
                                n272 = Wait (ms)(milliseconds to wait=u32 500) -> ()  [unwired: 1 out]
                                }
                                frame #2 {
                                n273 = property on="Load parameters" class="Bool (strict)"("Val(Sgnl)"=TRUE ("Value (Signaling)")) -> ()  [unwired: 2 in, 2 out]
                                n274 = case shown="True" "Green ON During Raster" {
                                frame False {
                                }
                                frame True {
                                n275 = property on="Green Laser ON" class="Bool (strict)"("Val(Sgnl)"=TRUE ("Value (Signaling)")) -> ()  [unwired: 2 in, 2 out]
                                }
                                }
                                }
                                frame #3 {
                                n276 = Wait (ms)(milliseconds to wait=u32 500) -> ()  [unwired: 1 out]
                                }
                                frame #4 {
                                n277 = property on="Trap Raster Scan" class="Bool (strict)"("Val(Sgnl)"=TRUE ("Value (Signaling)")) -> ()  [unwired: 2 in, 2 out]
                                }
                                frame #5 {
                                n278 = Wait (ms)(milliseconds to wait=u32 2000) -> ()  [unwired: 1 out]
                                }
                                frame #6 {
                                n279 = flat-sequence {
                                tunnel: w501 -> [w508]
                                frame #0 {
                                n280 = while {
                                stop <- w504 stop-if-true
                                n281 = local read "Raster Scanning..."() -> (w503:bool)
                                n282 = local read "Saving..."() -> (w506:bool)
                                n283 = Wait (ms)(milliseconds to wait=u32 100) -> ()  [unwired: 1 out]
                                n284 = Not(x=w506) -> (.not. x?=w505:bool)
                                n285 = Not(x=w503) -> (.not. x?=w502:bool)
                                n286 = And(x=w505, y=w502) -> (x .and. y?=w504:bool)
                                }
                                }
                                frame #1 {
                                n287 = local read "Tether"() -> (w509:bool)
                                n288 = case shown="True" w509 {
                                tunnel: w508 -> [_ w511]
                                frame False {
                                n289 = property on="Fish for Tether" class="Bool (strict)"("Val(Sgnl)"="Fish again after \nraster break?") -> ()  [unwired: 2 in, 2 out]
                                }
                                frame True {
                                n290 = stacked-sequence {
                                tunnel: w511 -> [_ w515 _ _]
                                frame #0 {
                                n291 = property on="Trap Delta (MHz)" class="DigNum (strict)"("Val(Sgnl)"="Move to Delta 2 (MHz)") -> ()  [unwired: 2 in, 2 out]
                                n292 = case shown="True" "Flow ON after\ntether testing?" {
                                frame False {
                                }
                                frame True {
                                n293 = property on="Sample Channel\nFlow" class="Bool (strict)"("Val(Sgnl)"=TRUE ("Value (Signaling)")) -> ()  [unwired: 2 in, 2 out]
                                }
                                }
                                }
                                frame #1 {
                                n294 = flat-sequence {
                                tunnel: w515 -> [w517]
                                frame #0 {
                                n295 = Wait (ms)(milliseconds to wait=u32 500) -> ()  [unwired: 1 out]
                                }
                                frame #1 {
                                n296 = case shown="\"6\"" w517 {
                                frame Default {
                                }
                                frame "6" {
                                n297 = property on="Green Laser ON" class="Bool (strict)"("Val(Sgnl)"=TRUE ("Green Laser ON/Interlacing")) -> ()  [unwired: 2 in, 2 out]
                                }
                                }
                                }
                                frame #2 {
                                n298 = Wait (ms)(milliseconds to wait=u32 500) -> ()  [unwired: 1 out]
                                }
                                frame #3 {
                                n299 = local write "Start Saving"("Save at end (5, 6)") -> ()
                                }
                                }
                                }
                                frame #2 {
                                n300 = local read "Bead Sep. Int. Time (s)"() -> (w523:dbl)
                                n301 = Multiply(x=w523, y=1000.0) -> (x*y=w522:dbl)
                                n302 = Wait (ms)(milliseconds to wait=w522) -> ()  [unwired: 1 out]
                                }
                                frame #3 {
                                n303 = property on="Remove Offset" class="Bool (strict)"("Val(Sgnl)"=TRUE ("Value (Signaling)")) -> ()  [unwired: 2 in, 2 out]
                                }
                                }
                                }
                                }
                                }
                                }
                                }
                                }
                                }
                                frame "2", Default {
                                }
                              }
                            }
                          }
                        }
                      }
                      "Tether" <- "Tether Alarm?"
                    }
                  }
                }
                frame #2 {
                  n304 = local read "Oscillate Set 1"() -> (w530:bool)
                  n305 = local read "Stop All"() -> (w528:bool)
                  n306 = Or(x=w530, y=w525) -> (x .or. y?=w527:bool)
                  n307 = Not(x=w527) -> (.not. x?=w529:bool)
                  n308 = Compound Arithmetic op=OR(w528, w529) -> (w526:bool)
                }
              }
              n309 = node-c288() -> ()  [unwired: 2 out]
            }
            n310 = node-c288(w371) -> ()  [unwired: 1 out]
          }
        }
      }
      event "Fl. Triggered...": Value Change {
        n311 = event-data() -> ()  [unwired: 7 out]
        n312 = case shown="True" "Fl. Triggered..." {
          frame False {
          }
          frame True {
            n313 = node-c288() -> (w541:T21)  [unwired: 4 out]
            n314 = timed-loop {
              timing: w541 -> [_]
              timing-out: [_] -> w540
              tunnel: "Action" -> [w549]
              shift-right: [w546] -> _
              shift-left: u8 255 -> [w548]
              shift-right: [w543] -> _
              shift-left: 255 -> [w545]
              stop <- w542 stop-if-true
              # "Reset confocal spot"
              n315 = node-c288() -> ()  [unwired: 2 out]
              n316 = flat-sequence {
                tunnel: w549 -> [w569]
                tunnel: w548 -> [w568]
                tunnel: [w567] -> w547
                tunnel: w545 -> [w554]
                tunnel: [w553] -> w544
                tunnel: [w948] -> w542
                tunnel: w547 -> [w947]
                tunnel: [w947] -> w546
                tunnel: [w946] -> w543
                tunnel: w544 -> [w946]
                frame #0 {
                  n317 = local read "Delta Fl. 2"() -> (w566:dbl)
                  n318 = local read "Delta Fl. 1"() -> (w561:dbl)
                  n319 = Multiply(x="Fl. Delta Thresh. (kHz)", y=1000.0) -> (x*y=w556:dbl)
                  n320 = Select(t=w561, s="APD to Watch", f=w566) -> (s? t:f=w557:dbl)
                  n321 = Greater?(x=w557, y=w556) -> (0:w562:bool)
                  n322 = Or(x="Force Yank", y=w562) -> (x .or. y?=w560:bool)
                  n323 = And(x=w560, y="Yank when?") -> (x .and. y?=w558:bool)
                  n324 = case shown="False" w558 {
                    tunnel: w569 -> [w572 w773]
                    tunnel: w568 -> [w574 w769]
                    tunnel: [w574 w767] -> w567
                    tunnel: w557 -> [w580 _]
                    tunnel: w556 -> [w579 _]
                    tunnel: "Force Yank" -> [w577 _]
                    tunnel: w554 -> [w576 w766]
                    tunnel: [w575 w766] -> w553
                    frame False {
                      n325 = Negate(x=w579) -> (-x=w571:dbl)
                      n326 = local write "Fl. High"(TRUE ("Fl. High")) -> ()
                      n327 = Less?(x=w580, y=w571) -> (x < y?=w578:bool)
                      n328 = Or(x=w577, y=w578) -> (x .or. y?=w573:bool)
                      n329 = case shown="True" w573 {
                        tunnel: w576 -> [w581 w591]
                        tunnel: [w581 w590] -> w575
                        tunnel: w572 -> [_ w589]
                        frame False {
                        }
                        frame True {
                          n330 = flat-sequence {
                            tunnel: w591 -> [w597]
                            tunnel: w589 -> [w594]
                            tunnel: [w596] -> w588
                            tunnel: [w595] -> w587
                            tunnel: [w594] -> w586
                            tunnel: w585 -> [w593]
                            tunnel: [w593] -> w584
                            tunnel: w583 -> [w592]
                            tunnel: [w592] -> w582
                            tunnel: [w668] -> w590
                            tunnel: w588 -> [w668]
                            tunnel: w587 -> [w667]
                            tunnel: w586 -> [w666]
                            tunnel: w584 -> [w665]
                            tunnel: w582 -> [w664]
                            frame #0 {
                              n331 = call <vilib>:"Beep.vi"() -> ()  [unwired: 12 in]
                              n332 = local write "Waiting"(FALSE ("Waiting")) -> ()
                              n333 = Increment(x=w597) -> (x+1=w596:i32)
                              n334 = case shown="\"Image\"" w594 {
                                tunnel: w596 -> [_ w602 _]
                                frame "Alarm", Default {
                                }
                                frame "Yank" {
                                n335 = flat-sequence {
                                tunnel: w602 -> [w605]
                                tunnel: [w604] -> w601
                                tunnel: [w603] -> w600
                                tunnel: w601 -> [w615]
                                tunnel: w600 -> [w616]
                                frame #0 {
                                n336 = local read "Yank Delay (s)"() -> (w608:dbl)
                                n337 = local read "N Array El"() -> (w603:u8)
                                n338 = Quotient & Remainder(x=w605, y=w603) -> (x-y*floor(x/y)=w604:i32)  [unwired: 1 out]
                                n339 = Multiply(x=w608, y=1000.0) -> (x*y=w606:dbl)
                                n340 = Wait (ms)(milliseconds to wait=w606) -> ()  [unwired: 1 out]
                                }
                                frame #1 {
                                n341 = local read "Yank to which?"() -> (w610:bool)
                                n342 = local read "Random Choice"() -> (w620:bool)
                                n343 = local read "Yank to Trap Delta (MHz)"() -> (w613:dbl[])
                                n344 = local read "Yank to SP"() -> (w614:dbl[])
                                n345 = Random Number (0-1)() -> (number: 0 to 1=w619:dbl)
                                n346 = Multiply(x=w616, y=w619) -> (x*y=w618:dbl)
                                n347 = Round Toward -Infinity(1:w618) -> (0:w617:dbl)
                                n348 = Select(t=w617, s=w620, f=w615) -> (s? t:f=w611:dbl)
                                n349 = Select(t=w613, s=w610, f=w614) -> (s? t:f=w612:dbl[])
                                n350 = Index Array(array=w612, index=w611) -> (element=w609:dbl)
                                n351 = case shown="True" w610 {
                                tunnel: w609 -> [w621 w648]
                                frame False {
                                n352 = flat-sequence {
                                tunnel: w621 -> [w622]
                                frame #0 {
                                n353 = property on="Trap Pos FB SP" class="DigNum (strict)"("Val(Sgnl)"=w622) -> ()  [unwired: 2 in, 2 out]
                                }
                                frame #1 {
                                n354 = Wait (ms)(milliseconds to wait=u32 700) -> ()  [unwired: 1 out]
                                }
                                frame #2 {
                                n355 = local read "Action (%)"() -> (w627:dbl)
                                n356 = Absolute Value(x=w627) -> (abs(x)=w626:dbl)
                                n357 = Greater?(x=w626, y=70.0) -> (0:w624:bool)
                                n358 = property on="Remove Action Offset" class="Bool (strict)"("Val(Sgnl)"=w624) -> ()  [unwired: 2 in, 2 out]